vi "UHR-Fleezers Control (host) - 10.8MV_trial1.vi"() -> ()   [LabVIEW 2010] (continued)
    n1529 = Or(x=w5608, y=w5604) -> (x .or. y?=w5605:bool)
    n1530 = Square Root(x=w5388) -> (sqrt(x)=w5387:dbl)
    n1531 = Equal?(x="Tab Control 6", y=T37."High Res Display") -> (x = y?=w5528:bool)
    n1532 = Multiply(x="APD Disp. Scale", y=w5478) -> (x*y=w5487:waveform(dbl)[])
    n1533 = Multiply(x="APD Disp. Downsample", y=w5485) -> (x*y=w5483:dbl)
    n1534 = Multiply(x=10.0, y=w5387) -> (x*y=→"Trap 1 Position RMS (A)":dbl)
    n1535 = Divide(x=w5487, y=w5483) -> (x/y=w5455:waveform(dbl)[])
    n1536 = Index Array(array=w5455, index=0) -> (element=w5465:waveform(dbl))
    n1537 = case "For computing FFTs for display" shown="True" "Compute FFT" {
      tunnel: w5482 -> [_ w7808]
      frame False {
      }
      frame True {
        n1538 = Build Array("FFT 1 Choice 1", "FFT 1 Choice 2", "FFT 2 Choice 1", "FFT 2 Choice 2") -> (w7801:u16[])
        n1539 = Array Size(array=w7808) -> (size(s)=w7807:i32)
        n1540 = feedback-in #6(w7801) -> ()
        n1541 = feedback #6(u16[] [100, 100, 100, 100]) -> (w7802:u16[])
        n1542 = feedback-in #7("# Spectra to Ave.") -> ()
        n1543 = feedback #7("# Spectra to Ave.") -> (w7799:dbl)
        n1544 = Not Equal?(x="# Spectra to Ave.", y=w7799) -> (x != y?=w7798:bool)
        n1545 = Not Equal?(x=w7801, y=w7802) -> (x != y?=w7800:bool)
        n1546 = feedback #8(1.0) -> (w7785:dbl)
        n1547 = Compound Arithmetic op=OR("Reset FFT", w7800, w7798) -> (w7783:bool)
        n1548 = Select(t=1.0, s=w7783, f=w7785) -> (s? t:f=w7787:dbl)
        n1549 = Greater?(x=w7787, y="# Spectra to Ave.") -> (0:w7806:bool)
        n1550 = Increment(x=w7787) -> (x+1=w7786:dbl)
        n1551 = feedback-in #8(w7786) -> ()
        n1552 = local read "DMA Update Period (s)"() -> (w7781:dbl)
        n1553 = Multiply(x="# Spectra to Ave.", y=w7781) -> (x*y=→"Ave. Time (s)":dbl)
        n1554 = Build Array(cluster{"f0":dbl, "df":dbl, "magnitude":dbl[]} {"f0"=0.0, "df"=0.0, "magnitude"=[]} ("PSD")) -> (w7790:cluster{"f0":dbl, "df":dbl, "magnitude":dbl[]}[])
        n1555 = Build Array(w7790, w7790, w7790, w7790) -> (w7792:T49)
        n1556 = feedback #9(w7792) -> (w7797:T49)
        n1557 = for {
          N: 4 -> [_]
          tunnel: w7801 -> [w7830] mode=indexing
          tunnel: w7808 -> [w7831]
          tunnel: w7807 -> [w7833]
          tunnel: w7783 -> [w7826]
          tunnel: w7806 -> [w7825]
          tunnel: "# Spectra to Ave." -> [w7824]
          tunnel: [w7823] -> w7796 mode=indexing
          tunnel: w7797 -> [w7828] mode=indexing
          tunnel: [w7827] -> w7784 mode=indexing
          tunnel: w7787 -> [w7822]
          n1558 = Less?(x=w7830, y=w7833) -> (x < y?=w7832:bool)
          n1559 = Index Array(array=w7831, index=w7830) -> (element=w7829:waveform(dbl))
          n1560 = case shown="True" w7832 {
            tunnel: w7829 -> [_ w7850]
            tunnel: w7828 -> [w7835 w7848]
            tunnel: [w7835 w7836] -> w7827
            tunnel: w7826 -> [_ w7847]
            tunnel: w7825 -> [_ w7840]
            tunnel: w7824 -> [_ w7839]
            tunnel: [cluster{"f0":dbl, "df":dbl, "magnitude":dbl[]} {"f0"=0.0, "df"=0.0, "magnitude"=[]} ("PSD") w7841] -> w7823
            tunnel: w7822 -> [_ w7838]
            frame False {
            }
            frame True {
              n1561 = call <vilib>:"Std Deviation and Variance.vi"("X"=w7850) -> ("mean"=w7851:dbl)  [unwired: 1 in, 2 out]
              n1562 = Subtract(x=w7850, y=w7851) -> (x-y=w7849:waveform(dbl))
              n1563 = xnode "Spectral Measurements"("Signals"=w7849) -> ("PSD"=w7843:cluster{"f0":dbl, "df":dbl, "magnitude":dbl[]})  [unwired: 1 in, 1 out]
              n1564 = case shown="False" w7847 {
                tunnel: w7848 -> [w7860 _]
                tunnel: [w7856 w7865] -> w7836
                tunnel: w7843 -> [w7859 w7866]
                tunnel: w7840 -> [w7858 _]
                frame False {
                  n1565 = Build Array (concatenate)(w7860, w7859) -> (w7857:cluster{"f0":dbl, "df":dbl, "magnitude":dbl[]}[])
                  n1566 = case shown="True" w7858 {
                    tunnel: w7857 -> [w7861 w7864]
                    tunnel: [w7861 w7862] -> w7856
                    frame False {
                    }
                    frame True {
                      n1567 = Delete From Array(array=w7864, index=0) -> (array with subset deleted=w7862:cluster{"f0":dbl, "df":dbl, "magnitude":dbl[]}[])  [unwired: 1 in, 1 out]
                    }
                  }
                }
                frame True {
                  n1568 = Build Array(w7866) -> (w7865:cluster{"f0":dbl, "df":dbl, "magnitude":dbl[]}[])
                }
              }
              n1569 = for {
                tunnel: w7836 -> [w7855] mode=indexing
                tunnel: [w7854] -> w7846 mode=indexing
                workers-P: _ -> [_]
                n1570 = Unbundle By Name(w7855) -> ("magnitude"=w7854:dbl[])
              }
              n1571 = Transpose 2D Array(2D array=w7846) -> (transposed array=w7845:dbl[][])
              n1572 = for {
                tunnel: w7845 -> [w7853] mode=indexing
                tunnel: [w7852] -> w7844 mode=indexing
                workers-P: _ -> [_]
                n1573 = Add Array Elements(numeric array=w7853) -> (sum=w7852:dbl)
              }
              n1574 = Select(t=w7839, s=w7840, f=w7838) -> (s? t:f=w7837:dbl)
              n1575 = Divide(x=w7844, y=w7837) -> (x/y=w7842:dbl[])
              n1576 = Bundle By Name(cluster=w7843, "magnitude"=w7842) -> (w7841:cluster{"f0":dbl, "df":dbl, "magnitude":dbl[]})
            }
          }
        }
        n1577 = case shown="True" w7783 {
          tunnel: w7784 -> [w7815 w7821]
          tunnel: [w7815 w7816] -> w7782
          frame False {
          }
          frame True {
            n1578 = Array Subset(array=w7821, index (row)=0 ("index"), length (row)=4 ("length"), index (col)=0 ("index"), length (col)=1 ("length")) -> (w7816:T49)
          }
        }
        n1579 = feedback-in #9(w7782) -> ()
        n1580 = Split 1D Array(array=w7796, index=2) -> (first subarray=→"FFT 1":cluster{"f0":dbl, "df":dbl, "magnitude":dbl[]}[], second subarray=→"FFT 2":cluster{"f0":dbl, "df":dbl, "magnitude":dbl[]}[])
      }
    }
    n1581 = Index Array(array=w5455, index=1) -> (element=w5463:waveform(dbl))
    n1582 = case "For displaying the high resolution display (no downsampling)" shown="True" w5528 {
      tunnel: w5482 -> [_ w5990]
      frame False {
      }
      frame True {
        n1583 = Index Array(array=w5990, index="High Res. Display") -> (element=w5991:waveform(dbl))
        n1584 = call <vilib>:"Std Deviation and Variance.vi"("X"=w5991) -> ("mean"=w5998:dbl, "standard deviation"=w6003:dbl)  [unwired: 1 in, 1 out]
        "Mean Intensity" <- w5998
        "Sigma" <- w6003
        n1585 = Subtract(x=w5991, y=w5998) -> (x-y=w5997:waveform(dbl))
        n1586 = Select(t=w5997, s="Subtract mean", f=w5991) -> (s? t:f=→"1 Channel":waveform(dbl))
        n1587 = Divide(x=w6003, y=w5998) -> (x/y=→"Sigma/Mean":dbl)
        n1588 = feedback #10(1) -> (w5992:i32)
        n1589 = Greater Or Equal?(x=w5992, y="Slow mean N ave.") -> (x >= y?=w6005:bool)
        n1590 = Increment(x=w5992) -> (x+1=w6007:i32)
        n1591 = Select(t=1, s=w6005, f=w6007) -> (s? t:f=w5994:i32)
        n1592 = feedback-in #10(w5994) -> ()
        n1593 = feedback #11() -> (w5995:waveform(dbl))  [unwired: 1 out]
        n1594 = case shown="Default" w5992 {
          tunnel: [w6010 w6013] -> w5996
          tunnel: w5995 -> [w6012 _]
          tunnel: w5991 -> [w6011 w6013]
          frame Default {
            n1595 = call-poly <vilib>:"Append Waveforms.vi"("waveform B"=w6011, "waveform A"=w6012) -> ("waveform out"=w6010:waveform(dbl))  [unwired: 1 in, 8 out]
          }
          frame 1 {
          }
        }
        n1596 = feedback-in #11(w5996) -> ()
        n1597 = case shown="True" w6005 {
          tunnel: w5996 -> [_ w6009]
          frame False {
          }
          frame True {
            n1598 = call <vilib>:"Mean.vi"("X"=w6009) -> ("mean"=→"Slow mean":dbl)  [unwired: 1 out]
          }
        }
      }
    }
    n1599 = case "For plotting results of scanning MCL" shown="True" w5605 {
      tunnel: w5604 -> [_ w6521]
      tunnel: w5521 -> [_ w6617]
      tunnel: w5613 -> [_ _]
      tunnel: w5482 -> [_ w6591]
      tunnel: w5457 -> [_ w6522]
      tunnel: w5456 -> [_ w6495]
      frame False {
      }
      frame True {
        w6502 = u32 0 items=["Horizontal", "Vertical", "Central", "1st Diagonal", "2nd Diagonal"] ("Type of Symmetry")
        w6530 = u32 0 items=["Horizontal", "Vertical", "Central", "1st Diagonal", "2nd Diagonal"] ("Type of Symmetry")
        w6533 = u32 0 items=["Horizontal", "Vertical", "Central", "1st Diagonal", "2nd Diagonal"] ("Type of Symmetry")
        w6562 = u32 0 items=["Horizontal", "Vertical", "Central", "1st Diagonal", "2nd Diagonal"] ("Type of Symmetry")
        n1600 = Index Array(array=w6591, index=10) -> (element=w6597:waveform(dbl))
        n1601 = Index Array(array=w6591, index=11) -> (element=w6594:waveform(dbl))
        n1602 = local read "Cycles/step (MCL)"() -> (w6547:u64)
        n1603 = Index Array(array=w6591, index="Channel") -> (element=w6593:waveform(dbl))
        n1604 = Unbundle(w6495) -> ("New Image"=w6494:T2, "New Image"=w6493:T2, "New Image"=w6492:T2, "New Image"=w6491:T2)
        n1605 = Unbundle By Name(w6597) -> ("Y"=w6549:dbl[])
        n1606 = Unbundle By Name(w6594) -> ("Y"=w6551:dbl[])
        n1607 = Unbundle By Name(w6593) -> ("Y"=w6556:dbl[])
        n1608 = call "downsample 1D array - double.vi"("Ave N"=w6547, "Array In"=w6549) -> ("Array Out"=w6548:dbl[])  [unwired: 1 out]
        n1609 = call "downsample 1D array - double.vi"("Ave N"=w6547, "Array In"=w6551) -> ("Array Out"=w6550:dbl[])  [unwired: 1 out]
        n1610 = call "downsample 1D array - double.vi"("Ave N"=w6547, "Array In"=w6556) -> ("Array Out"=w6555:dbl[])  [unwired: 1 out]
        n1611 = feedback #12(w6617) -> (w6618:dbl[])
        n1612 = Build Array (concatenate)(w6618, w6617) -> (w6599:dbl[])
        n1613 = feedback #13(w6522) -> (w6524:dbl[])
        n1614 = Build Array (concatenate)(w6524, w6522) -> (w6523:dbl[])
        n1615 = local read "Scan steps (MCL)"() -> (w6504:u64)
        n1616 = Select(t=w6617, s=w6521, f=w6599) -> (s? t:f=w6603:dbl[])
        n1617 = feedback-in #12(w6603) -> ()
        n1618 = Select(t=w6522, s=w6521, f=w6523) -> (s? t:f=w6505:dbl[])
        n1619 = feedback-in #13(w6505) -> ()
        n1620 = local read "Scan lines (y)"() -> (w6490:u64)
        n1621 = local read "N APD Samp/step"() -> (w6506:dbl)
        n1622 = feedback #14(w6548) -> (w6605:dbl[])
        n1623 = Build Array (concatenate)(w6605, w6548) -> (w6596:dbl[])
        n1624 = feedback #15(w6555) -> (w6615:dbl[])
        n1625 = Build Array (concatenate)(w6615, w6555) -> (w6614:dbl[])
        n1626 = feedback #16(w6550) -> (w6607:dbl[])
        n1627 = Build Array (concatenate)(w6607, w6550) -> (w6608:dbl[])
        n1628 = Select(t=w6548, s=w6521, f=w6596) -> (s? t:f=w6552:dbl[])
        n1629 = feedback-in #14(w6552) -> ()
        n1630 = Select(t=w6555, s=w6521, f=w6614) -> (s? t:f=w6554:dbl[])
        n1631 = feedback-in #15(w6554) -> ()
        n1632 = Select(t=w6550, s=w6521, f=w6608) -> (s? t:f=w6553:dbl[])
        n1633 = feedback-in #16(w6553) -> ()
        n1634 = Multiply(x=w6504, y=u64 2) -> (x*y=w6489:u64)
        n1635 = call "integrate 1D array interval - double.vi"("Ave N"=w6506, "Array In"=w6505) -> ("Array Out"=w6517:dbl[])  [unwired: 1 out]
        n1636 = call "integrate 1D array interval - double.vi"("Ave N"=w6506, "Array In"=w6603) -> ("Array Out"=w6602:dbl[])  [unwired: 1 out]
        n1637 = Array Size(array=w6517) -> (size(s)=w6518:i32)
        n1638 = Array Size(array=w6602) -> (size(s)=w6604:i32)
        n1639 = Multiply(x=w6490, y=w6489) -> (x*y=w6520:u64)
        n1640 = Multiply(x=w6490, y=w6489) -> (x*y=w6612:u64)
        n1641 = call <vilib>:"Mean.vi"("X"=w6552) -> ("mean"=w6536:dbl)  [unwired: 1 out]
        n1642 = Subtract(x=w6520, y=w6518) -> (x-y=w6511:u64)
        n1643 = call <vilib>:"Mean.vi"("X"=w6554) -> ("mean"=w6541:dbl)  [unwired: 1 out]
        n1644 = call <vilib>:"Mean.vi"("X"=w6553) -> ("mean"=w6539:dbl)  [unwired: 1 out]
        n1645 = call <vilib>:"Mean.vi"("X"=w6517) -> ("mean"=w6508:dbl)  [unwired: 1 out]
        n1646 = Subtract(x=w6612, y=w6604) -> (x-y=w6546:u64)
        n1647 = call <vilib>:"Mean.vi"("X"=w6602) -> ("mean"=w6543:dbl)  [unwired: 1 out]
        n1648 = Initialize Array(1.0 ("element"), w6511) -> (w6507:dbl[])
        n1649 = Initialize Array(1.0 ("element"), w6546) -> (w6537:dbl[])
        n1650 = Multiply(x=w6507, y=w6508) -> (x*y=w6509:dbl[])
        n1651 = Multiply(x=w6537, y=w6539) -> (x*y=w6540:dbl[])
        n1652 = Multiply(x=w6537, y=w6541) -> (x*y=w6542:dbl[])
        n1653 = Multiply(x=w6537, y=w6536) -> (x*y=w6538:dbl[])
        n1654 = Multiply(x=w6537, y=w6543) -> (x*y=w6544:dbl[])
        n1655 = Build Array (concatenate)(w6552, w6538) -> (w6606:dbl[])
        n1656 = Build Array (concatenate)(w6554, w6542) -> (w6610:dbl[])
        n1657 = Build Array (concatenate)(w6553, w6540) -> (w6609:dbl[])
        n1658 = Build Array (concatenate)(w6517, w6509) -> (w6519:dbl[])
        n1659 = Build Array (concatenate)(w6602, w6544) -> (w6611:dbl[])
        n1660 = Reshape Array(w6606, w6490, w6489) -> (w6572:dbl[][])
        n1661 = Reshape Array(w6519, w6490, w6489) -> (w6515:dbl[][])
        n1662 = Reshape Array(w6610, w6490, w6489) -> (w6564:dbl[][])
        n1663 = Reshape Array(w6609, w6490, w6489) -> (w6579:dbl[][])
        n1664 = Reshape Array(w6611, w6490, w6489) -> (w6589:dbl[][])
        n1665 = Array Subset(array=w6579, index (col)=0 ("index"), length (col)=w6504) -> (w6584:dbl[][])  [unwired: 2 in]
        n1666 = Array Subset(array=w6579, index (col)=w6504) -> (w6582:dbl[][])  [unwired: 3 in]
        n1667 = Array Subset(array=w6564, index (col)=0 ("index"), length (col)=w6504) -> (w6570:dbl[][])  [unwired: 2 in]
        n1668 = Array Subset(array=w6564, index (col)=w6504) -> (w6568:dbl[][])  [unwired: 3 in]
        n1669 = Array Subset(array=w6515, index (col)=0 ("index"), length (col)=w6504) -> (w6514:dbl[][])  [unwired: 2 in]
        n1670 = Array Subset(array=w6515, index (col)=w6504) -> (w6512:dbl[][])  [unwired: 3 in]
        n1671 = Array Subset(array=w6589, index (col)=0 ("index"), length (col)=w6504) -> (w6588:dbl[][])  [unwired: 2 in]
        n1672 = Array Subset(array=w6589, index (col)=w6504) -> (w6586:dbl[][])  [unwired: 3 in]
        n1673 = Array Subset(array=w6572, index (col)=0 ("index"), length (col)=w6504) -> (w6577:dbl[][])  [unwired: 2 in]
        n1674 = Array Subset(array=w6572, index (col)=w6504) -> (w6575:dbl[][])  [unwired: 3 in]
        n1675 = for {
          tunnel: w6584 -> [w6626] mode=indexing
          tunnel: [w6625] -> w6583 mode=indexing
          workers-P: _ -> [_]
          n1676 = Reverse 1D Array(array=w6626) -> (reversed array=w6625:dbl[])
        }
        n1677 = for {
          tunnel: w6570 -> [w6622] mode=indexing
          tunnel: [w6621] -> w6569 mode=indexing
          workers-P: _ -> [_]
          n1678 = Reverse 1D Array(array=w6622) -> (reversed array=w6621:dbl[])
        }
        n1679 = for {
          tunnel: w6514 -> [w6620] mode=indexing
          tunnel: [w6619] -> w6513 mode=indexing
          workers-P: _ -> [_]
          n1680 = Reverse 1D Array(array=w6620) -> (reversed array=w6619:dbl[])
        }
        n1681 = for {
          tunnel: w6588 -> [w6628] mode=indexing
          tunnel: [w6627] -> w6587 mode=indexing
          workers-P: _ -> [_]
          n1682 = Reverse 1D Array(array=w6628) -> (reversed array=w6627:dbl[])
        }
        n1683 = for {
          tunnel: w6577 -> [w6624] mode=indexing
          tunnel: [w6623] -> w6576 mode=indexing
          workers-P: _ -> [_]
          n1684 = Reverse 1D Array(array=w6624) -> (reversed array=w6623:dbl[])
        }
        n1685 = Index Array(array=w6589, index (row)=0) -> (element=→"Waveform Graph":dbl[])  [unwired: 1 in]
        n1686 = Add(x=w6583, y=w6582) -> (x+y=w6581:dbl[][])
        n1687 = Add(x=w6569, y=w6568) -> (x+y=w6567:dbl[][])
        n1688 = Add(x=w6513, y=w6512) -> (x+y=w6497:dbl[][])
        n1689 = Add(x=w6587, y=w6586) -> (x+y=w6561:dbl[][])
        n1690 = Add(x=w6576, y=w6575) -> (x+y=w6574:dbl[][])
        n1691 = Divide(x=w6567, y=2) -> (x/y=w6565:dbl[][])
        n1692 = Divide(x=w6581, y=2) -> (x/y=w6526:dbl[][])
        n1693 = Divide(x=w6574, y=2) -> (x/y=w6528:dbl[][])
        n1694 = To Single Precision Float(number=w6561) -> (single precision float=w6560:sgl[][])
        n1695 = Transpose 2D Array(2D array=w6565) -> (transposed array=→"Data map":dbl[][])
        n1696 = To Single Precision Float(number=w6497) -> (single precision float=w6501:sgl[][])
        n1697 = To Single Precision Float(number=w6526) -> (single precision float=w6532:sgl[][])
        n1698 = To Single Precision Float(number=w6528) -> (single precision float=w6529:sgl[][])
        n1699 = call "IMAQ ArrayToImage"("Image Pixels (Float)"=w6560, "Image"=w6494) -> ("Image Out"=w6563:T2)  [unwired: 8 in, 1 out]
        n1700 = call "IMAQ ArrayToImage"("Image Pixels (Float)"=w6501, "Image"=w6493) -> ("Image Out"=w6503:T2)  [unwired: 8 in, 1 out]
        n1701 = call "IMAQ ArrayToImage"("Image Pixels (Float)"=w6532, "Image"=w6492) -> ("Image Out"=w6534:T2)  [unwired: 8 in, 1 out]
        n1702 = call "IMAQ ArrayToImage"("Image Pixels (Float)"=w6529, "Image"=w6491) -> ("Image Out"=w6531:T2)  [unwired: 8 in, 1 out]
        n1703 = call "IMAQ Symmetry"("Type of Symmetry"=w6562, "Image Src"=w6563) -> ("Image Dst Out"=w6558:T2)  [unwired: 3 in, 1 out]
        n1704 = call "IMAQ Symmetry"("Type of Symmetry"=w6502, "Image Src"=w6503) -> ("Image Dst Out"=w6499:T2)  [unwired: 3 in, 1 out]
        n1705 = call "IMAQ Symmetry"("Type of Symmetry"=w6533, "Image Src"=w6534) -> ("Image Dst Out"=→"Detection Laser X":T2)  [unwired: 3 in, 1 out]
        n1706 = call "IMAQ Symmetry"("Type of Symmetry"=w6530, "Image Src"=w6531) -> ("Image Dst Out"=→"Detection Laser Y":T2)  [unwired: 3 in, 1 out]
        n1707 = call "IMAQ Set Simple Calibration"("Calibration Axis Info"=T38 {"Origin Pixel"={"X"=0.0, "Y"=0.0}, "Angle Relative to Horizontal (deg)"=0.0, "Axis Reference"=0}, "Grid Descriptor"=T39 {"X Step"=0.3, "Y Step"=0.3, "Unit"=enum."Undefined"}, "Image"=w6558) -> ("Calibrated Image"=→"APD 1":T2)  [unwired: 7 in, 1 out]
        n1708 = call "IMAQ Set Simple Calibration"("Calibration Axis Info"=T38 {"Origin Pixel"={"X"=0.0, "Y"=0.0}, "Angle Relative to Horizontal (deg)"=0.0, "Axis Reference"=0}, "Grid Descriptor"=T39 {"X Step"=0.3, "Y Step"=0.3, "Unit"=enum."Undefined"}, "Image"=w6499) -> ("Calibrated Image"=→"APD 2":T2)  [unwired: 7 in, 1 out]
      }
    }
    n1709 = Subtract(x=w5463, y="APD 2 Offset") -> (x-y=w5460:waveform(dbl))
    n1710 = Subtract(x=w5465, y="APD 1 Offset") -> (x-y=w5461:waveform(dbl))
    n1711 = Index Array(array=w5480, index=3) -> (element=w5549:waveform(dbl))
    n1712 = Index Array(array=w5480, index=6) -> (element=w5546:waveform(dbl))
    n1713 = Build Array(w5461, w5460) -> (→"APD Chart":waveform(dbl)[])
    n1714 = Array Size(array=w5538) -> (size(s)=w5593:i32)
    n1715 = call <vilib>:"Std Deviation and Variance.vi"("X"=w5473) -> ("standard deviation"=w5472:dbl)  [unwired: 1 in, 2 out]
    n1716 = Add Array Elements(numeric array=w5473) -> (sum=w5475:u32)
    n1717 = Add Array Elements(numeric array=w5538) -> (sum=w5603:u32)
    n1718 = call <vilib>:"Std Deviation and Variance.vi"("X"=w5538) -> ("standard deviation"=w5537:dbl)  [unwired: 1 in, 2 out]
    n1719 = Divide(x="T1 offset_x (mV)", y=1000.0) -> (x/y=w5550:dbl)
    n1720 = Divide(x=w5472, y=w5471) -> (x/y=w5468:dbl)
    "Rate sigma (Hz) 2" <- w5468
    n1721 = Multiply(x=w5471, y=w5593) -> (x*y=w5474:dbl)
    "Int. Time (s)" <- w5474
    n1722 = Divide(x=w5475, y=w5474) -> (x/y=w5469:dbl)
    "APD 2 Rate (Hz)" <- w5469
    n1723 = Divide(x=w5603, y=w5474) -> (x/y=w5535:dbl)
    "APD 1 Rate (Hz)" <- w5535
    n1724 = Divide(x=w5537, y=w5471) -> (x/y=w5536:dbl)
    "Rate sigma (Hz)" <- w5536
    n1725 = Divide(x=w5468, y=w5469) -> (x/y=→"Sigma/Mean 2":dbl)
    n1726 = Divide(x=w5536, y=w5535) -> (x/y=→"Sigma/Mean":dbl)
    n1727 = Divide(x="T2 offset_x (mV)", y=1000.0) -> (x/y=w5548:dbl)
    n1728 = case shown="1" "Calibration" {
      tunnel: "T1 alpha_x (nm/V)" -> [_ w6457 w6478]
      tunnel: "T1 kappa_x (pN/nm)" -> [_ _ w6468]
      tunnel: "T2 alpha_x (nm/V)" -> [_ w6456 w6476]
      tunnel: "T2 kappa_x (pN/nm)" -> [_ _ w6469]
      tunnel: w5549 -> [w6439 w6454 w6474]
      tunnel: w5546 -> [w6438 w6452 w6472]
      tunnel: [w6439 w6451 w6471] -> w5579
      tunnel: [w6438 w6450 w6470] -> w5578
      tunnel: ["T1 X (V)" ("Label.Text") "T1 X (nm)" ("Label.Text") "T1 X (pN)" ("Label.Text")] -> w5567
      tunnel: ["T2 X (V)" ("Label.Text") "T2 X (nm)" ("Label.Text") "T2 X (pN)" ("Label.Text")] -> w5566
      tunnel: ["Position (V)" ("Label.Text") "Position (nm)" ("Label.Text") "Force (pN)" ("Label.Text")] -> w5568
      tunnel: w5548 -> [_ w6442 w6461]
      tunnel: w5550 -> [_ w6445 w6463]
      tunnel: ["Mean (V)" ("Label.Text") "Mean (nm)" ("Label.Text") "Mean (pN)" ("Label.Text")] -> w5563
      tunnel: ["Difference (V)" ("Label.Text") "Difference (nm)" ("Label.Text") "Difference (pN)" ("Label.Text")] -> w5488
      frame 0, Default {
      }
      frame 1 {
        # "position"
        n1729 = Unbundle By Name(w6454) -> ("Y"=w6458:dbl[])
        n1730 = Unbundle By Name(w6452) -> ("Y"=w6443:dbl[])
        n1731 = Subtract(x=w6458, y=w6445) -> (x-y=w6446:dbl[])
        n1732 = Subtract(x=w6443, y=w6442) -> (x-y=w6444:dbl[])
        n1733 = Multiply(x=w6444, y=w6456) -> (x*y=w6453:dbl[])
        n1734 = Multiply(x=w6457, y=w6446) -> (x*y=w6455:dbl[])
        n1735 = Bundle By Name(cluster=w6452, "Y"=w6453) -> (w6450:waveform(dbl))
        n1736 = Bundle By Name(cluster=w6454, "Y"=w6455) -> (w6451:waveform(dbl))
      }
      frame 2 {
        # "force"
        n1737 = Unbundle By Name(w6474) -> ("Y"=w6479:dbl[])
        n1738 = Unbundle By Name(w6472) -> ("Y"=w6477:dbl[])
        n1739 = Subtract(x=w6477, y=w6461) -> (x-y=w6462:dbl[])
        n1740 = Subtract(x=w6479, y=w6463) -> (x-y=w6464:dbl[])
        n1741 = Compound Arithmetic op=MULTIPLY(w6462, w6476, w6469) -> (w6473:dbl[])
        n1742 = Compound Arithmetic op=MULTIPLY(w6468, w6478, w6464) -> (w6475:dbl[])
        n1743 = Bundle By Name(cluster=w6472, "Y"=w6473) -> (w6470:waveform(dbl))
        n1744 = Bundle By Name(cluster=w6474, "Y"=w6475) -> (w6471:waveform(dbl))
      }
    }
    n1745 = feedback-in #17("Calibration") -> ()
    n1746 = feedback #17(u16 1 ("Calibration")) -> (w5570:u16)
    n1747 = Not Equal?(x=w5570, y="Calibration") -> (x != y?=w5526:bool)
    n1748 = Unbundle By Name(w5549) -> ("Y"=w5552:dbl[])
    n1749 = Unbundle By Name(w5546) -> ("Y"=w5555:dbl[])
    n1750 = Subtract(x=w5552, y=w5550) -> (x-y=w5553:dbl[])
    n1751 = Subtract(x=w5555, y=w5548) -> (x-y=w5554:dbl[])
    n1752 = disable-structure shown="Enabled" {
      disable-tunnel: [-1.0 ("y") 1.0] -> w5556
      frame Disabled {
      }
      frame Enabled {
      }
    }
    n1753 = Multiply(x=w5554, y="T2 alpha_x (nm/V)") -> (x*y=w5545:dbl[])
    n1754 = Multiply(x="T1 alpha_x (nm/V)", y=w5553) -> (x*y=w5544:dbl[])
    n1755 = Multiply(x=w5578, y=w5556) -> (x*y=w5557:waveform(dbl))
    n1756 = case shown="True" "Read Lateness and Rel Phase" {
      tunnel: w5380 -> [w6014 w6036]
      tunnel: w5379 -> [w6015 w6035]
      tunnel: [w6014 w6034] -> w5541
      tunnel: [w6015 w6033] -> w5540
      frame False {
      }
      frame True {
        n1757 = xnode "Read/Write Control"("FPGA VI Reference In"=w6036, "error in"=w6035) -> ("FPGA VI Reference Out"=w6034:T19, "error out"=w6033:errorcluster, "GI Relative phase"=→"GI relative phase":i16, "Relative phase"=→"Relative phase (AI1)":i16, "AI Late Counter"=→"Late Counter (AI1)":u16, "GI Late Counter"=→"GI Late Counter":u16, "MCL Late Counter"=→"MCL Late Counter":u16, "MCL Relative Phase"=→"Relative Phase (MCL)":i16, "APD Acq Relative Phase"=→"APD Acq Relative Phase":i16, "APD 1 Gate Relative Phase"=→"APD 1 Gate Relative Phase":i16, "APD 2 Gate Relative Phase"=→"APD 2 Gate Relative Phase":i16, "APD Acq Late Counter"=→"APD Acq Late Counter":u16, "APD 1 Gate Late Counter"=→"APD 1 Gate Late Counter":u16, "APD 2 Gate Late Counter"=→"APD 2 Gate Late Counter":u16, "Green FB Relative Phase"=→"Relative phase (Green FB)":i16, "GI Relative phase 2"=→"GI relative phase 2":i16, "GI Late Counter 2"=→"GI Late Counter 2":u16, "Trap Pos FIFO Timeout"=→"Trap Pos FIFO Timeout":u16, "Trap AI FIFO Timeout"=→"Trap AI FIFO Timeout":u16)
      }
    }
    n1758 = Subtract(x=w5545, y=w5544) -> (x-y=w5543:dbl[])
    n1759 = Unbundle By Name(w5578) -> ("Y"=w5513:dbl[])
    n1760 = Unbundle By Name(w5579) -> ("Y"=w5514:dbl[])
    n1761 = Build Array(w5579, w5557) -> (→"Force":waveform(dbl)[])
    n1762 = Subtract(x=w5543, y="Offset (nm)") -> (x-y=w5511:dbl[])
    n1763 = call <vilib>:"Mean.vi"("X"=w5513) -> ("mean"=w5492:dbl)  [unwired: 1 out]
    "T2 X" <- w5492
    n1764 = Absolute Value(x=w5514) -> (abs(x)=w5515:dbl[])
    n1765 = Absolute Value(x=w5513) -> (abs(x)=w5516:dbl[])
    n1766 = call <vilib>:"Mean.vi"("X"=w5514) -> ("mean"=w5493:dbl)  [unwired: 1 out]
    "T1 X" <- w5493
    n1767 = Add(x=w5515, y=w5516) -> (x+y=w5517:dbl[])
    n1768 = Bundle By Name(cluster=w5549, "Y"=w5511) -> (w5479:waveform(dbl))
    "Bead Separation" <- w5479
    n1769 = Divide(x=w5517, y=2.0) -> (x/y=→"Vec Mean of T1 T2":dbl[])
    n1770 = case shown="True" w5526 {
      tunnel: w5568 -> [_ w6432]
      tunnel: w5567 -> [_ w6431]
      tunnel: w5566 -> [_ w6430]
      tunnel: w5563 -> [_ w6429]
      tunnel: w5488 -> [_ w6428]
      frame False {
      }
      frame True {
        n1771 = property on="Force" class="WFChart (strict)"("YScale.NameLbl.Text"=w6432) -> ()  [unwired: 2 in, 2 out]
        n1772 = property on="T2 X" class="DigNum (strict)"("Caption.Text"=w6430) -> ()  [unwired: 2 in, 2 out]
        n1773 = property on="T1 X" class="DigNum (strict)"("Caption.Text"=w6431) -> ()  [unwired: 2 in, 2 out]
        n1774 = property on="Mean" class="DigNum (strict)"("Caption.Text"=w6429) -> ()  [unwired: 2 in, 2 out]
        n1775 = property on="Difference" class="DigNum (strict)"("Caption.Text"=w6428) -> ()  [unwired: 2 in, 2 out]
      }
    }
    n1776 = local read "Tether"() -> (w5520:bool)
    n1777 = Absolute Value(x=w5493) -> (abs(x)=w5490:dbl)
    n1778 = Absolute Value(x=w5492) -> (abs(x)=w5489:dbl)
    n1779 = Add(x=w5490, y=w5489) -> (x+y=w5565:dbl)
    n1780 = Subtract(x=w5490, y=w5489) -> (x-y=→"Difference":dbl)
    n1781 = feedback #18(w5511) -> (w5510:dbl[])
    n1782 = Divide(x=w5565, y=2.0) -> (x/y=w5519:dbl)
    "Mean" <- w5519
    n1783 = case shown="True" w5520 {
      tunnel: w5519 -> [_ w5973]
      frame False {
      }
      frame True {
        n1784 = Greater?(x="Lost Tether Alarm Threshold (pN)", y=w5973) -> (0:w5971:bool)
        n1785 = case shown="True" w5971 {
          frame False {
          }
          frame True {
            n1786 = flat-sequence {
              frame #0 {
                # "stop only if saving"
                n1787 = local read "Saving..."() -> (w5986:bool)
                n1788 = And(x=w5986, y="TA Cancel Save?") -> (x .and. y?=w5985:bool)
                n1789 = local write "Stop Saving"(w5985) -> ()
              }
              frame #1 {
                n1790 = case shown="True" "TA Green Off?" {
                  frame False {
                  }
                  frame True {
                    w5989 = FALSE ("Fl. Triggered...")
                    n1791 = local write "Fl. Triggered..."(w5989) -> ()
                    n1792 = property on="Green Laser ON/Interlacing" class="Bool (strict)"("Val(Sgnl)"=w5989) -> ()  [unwired: 2 in, 2 out]
                  }
                }
              }
            }
            n1793 = local read "Time tether formed"() -> (w5980:timestamp)
            n1794 = Get Date/Time In Seconds() -> (seconds since 1Jan1904=w5981:timestamp)
            n1795 = Subtract(x=w5981, y=w5980) -> (x-y=w5979:dbl)
            n1796 = Number To Decimal String(number=w5979) -> (decimal integer string=w5976:string)  [unwired: 1 out]
            n1797 = local read "Messages"() -> (w5983:string)
            n1798 = call <vilib>:"Beep.vi"() -> ()  [unwired: 3 in, 9 out]
            n1799 = Concatenate Strings("Lost tether (" ("Message to add"), w5976, " s)." ("string")) -> (w5978:string)
            n1800 = local write "Tether"(FALSE ("Tether")) -> ()
            n1801 = call "Update messages.vi"("Message to add"=w5978, "Old message string"=w5983) -> ("New message string"=w5982:string)
            n1802 = local write "Messages"(w5982) -> ()
            n1803 = property on="Trap Pos. FB ON" class="Bool (strict)"("Val(Sgnl)"=FALSE ("Value (Signaling)")) -> ()  [unwired: 2 in, 2 out]
          }
        }
      }
    }
    n1804 = Build Array (concatenate)(w5511, w5510) -> (w5509:dbl[])
    n1805 = Split 1D Array(array=w5509, index=w5391) -> (first subarray=w5505:dbl[])  [unwired: 1 out]
    n1806 = feedback-in #18(w5505) -> ()
    n1807 = call <vilib>:"Mean.vi"("X"=w5505) -> ("mean"=w5504:dbl)  [unwired: 1 out]
    "Bead Mean (nm)" <- w5504
    n1808 = Subtract(x=w5505, y=w5504) -> (x-y=w5503:dbl[])
    n1809 = Square(x=w5503) -> (x^2=w5502:dbl[])
    n1810 = call <vilib>:"Mean.vi"("X"=w5502) -> ("mean"=w5501:dbl)  [unwired: 1 out]
    n1811 = Square Root(x=w5501) -> (sqrt(x)=w5500:dbl)
    n1812 = Multiply(x=10.0, y=w5500) -> (x*y=→"RMS (Ang)":dbl)
    n1813 = xnode "Read/Write Control"("FPGA VI Reference In"=w5541, "error in"=w5540) -> ("FPGA VI Reference Out"=w5659:T19, "error out"=w5653:errorcluster, "AI2 Y Sum Set 1"=w5649:i16, "AI2 Y Sum Set 2"=w5648:i16, "AI1 X Set 1"=w5425:fxp<+/-,16,1>, "AI1 X Set 2"=w5424:fxp<+/-,16,1>, "Trap Pos FB Int Signal"=→"Trap Pos FB Int Signal":fxp<+/-,24,9>, "Trap Pos FB Int-Norm Signal"=→"Trap Pos FB Int-Norm Signal":fxp<+/-,16,1>, "Trap Pos FB Action"=w5418:i64, "Scanning"=→"AOD Scanning":bool, "Scan I"=→"AOD Scan I":u64, "Scanning MCL"=w5651:bool, "Scan I (MCL)"=→"MCL Scan I":u64, "Green FB Signals"=w5588:T43)  [unwired: 1 out]
    "MCL Scanning" <- w5651
    "Trap Pos FB Action" <- w5418
    n1814 = local read "AI2 (V)"() -> (w5650:cluster{"Set 1":dbl, "Set 2":dbl})
    n1815 = Bundle By Name(cluster=w5650, "Set 1"=w5649, "Set 2"=w5648) -> (w5646:cluster{"Set 1":dbl, "Set 2":dbl})
    n1816 = Divide(x=w5418, y=327.67) -> (x/y=→"Action (%)":dbl)
    n1817 = local read "Trap X (AI1)"() -> (w5438:T10)
    n1818 = Divide(x=w5646, y=3276.7) -> (x/y=w5645:cluster{"Set 1":dbl, "Set 2":dbl})
    n1819 = local write "AI2 (V)"(w5645) -> ()
    n1820 = Bundle(cluster=w5438, "Trap 1"=w5425, "Trap 2"=w5424) -> (→"Trap X (AI1)":T10)
    n1821 = Divide(x=w5588, y=3276.7) -> (x/y=w5584:T50)
    n1822 = Unbundle By Name(w5584) -> ("Green FB Ch 0"=w5587:dbl, "Green FB Ch 1"=w5586:dbl, "Green FB Ch 2"=w5585:dbl)
    n1823 = Divide(x=w5587, y=w5585) -> (x/y=w5583:dbl)
    n1824 = Divide(x=w5586, y=w5585) -> (x/y=w5582:dbl)
    n1825 = flat-sequence "To save data" {
      tunnel: [w8289] -> w5670
      tunnel: [w8290] -> w5669
      tunnel: w5619 -> [w8283]
      tunnel: w5507 -> [w8287]
      tunnel: ["Save Calibration"] -> w5642
      tunnel: w5639 -> [w8286]
      tunnel: [w8279] -> w5638
      tunnel: [w8276] -> w5637
      tunnel: [w8273] -> w5636
      tunnel: w5618 -> [w8275]
      tunnel: w5524 -> [w8269]
      tunnel: [w8269] -> w5523
      tunnel: ["Start Saving"] -> w5481
      tunnel: [w8263] -> w5407
      tunnel: [w8262] -> w5406
      tunnel: w5670 -> [w8524]
      tunnel: w5669 -> [w8523]
      tunnel: w5408 -> [w8522]
      tunnel: w5642 -> [w8521]
      tunnel: w5638 -> [w8519]
      tunnel: w5637 -> [w8518]
      tunnel: w5636 -> [w8517]
      tunnel: w5494 -> [w8516]
      tunnel: w5533 -> [w8515]
      tunnel: w5523 -> [w8514]
      tunnel: w5481 -> [w8513]
      tunnel: w5479 -> [w8512]
      tunnel: w5455 -> [w8511]
      tunnel: w5407 -> [w8510]
      tunnel: w5406 -> [w8509]
      tunnel: w5405 -> [w8508]
      frame #0 {
        n1826 = Or(x="Save N Sets", y="Start Saving") -> (x .or. y?=w8270:bool)
        n1827 = To Double Precision Float(number=w8286) -> (double precision float=w8280:dbl)
        n1828 = Build Array(w8270, "Save Calibration", w8283, w8275) -> (w8285:bool[])
        n1829 = Compound Arithmetic op=OR("Save Calibration", w8283, w8270, w8275) -> (w8288:bool)
        n1830 = Boolean Array To Number(Boolean array=w8285) -> (number=w8282:u32)
        n1831 = feedback #19(FALSE ("Save APD Data\nwith Trap Data")) -> (w8264:bool)
        n1832 = feedback #20(refnum<k0> refnum) -> (w8291:refnum<file>)
        n1833 = feedback #21(refnum<k0> refnum) -> (w8266:refnum<file>)
        n1834 = feedback #22(FALSE ("Save APD Data\nwith Trap Data")) -> (w8274:bool)
        n1835 = feedback #23(refnum<k0> refnum) -> (w8277:refnum<file>)
        n1836 = feedback #24(0) -> (w8293:i32)
        n1837 = feedback #25() -> (w8281:u32)  [unwired: 1 out]
        n1838 = case shown="True" w8288 {
          tunnel: [w8300 1] -> w8289
          tunnel: w8293 -> [w8302 _]
          tunnel: [w8301 w8320] -> w8290
          tunnel: w8291 -> [w8301 _]
          tunnel: w8287 -> [_ w8340]
          tunnel: w8280 -> [_ w8338]
          tunnel: w8282 -> [_ w8341]
          tunnel: [w8299 w8319] -> w8279
          tunnel: w8281 -> [w8299 _]
          tunnel: [w8298 w8317] -> w8276
          tunnel: w8277 -> [w8298 _]
          tunnel: [w8297 w8316] -> w8273
          tunnel: w8274 -> [w8297 _]
          tunnel: "Start Saving" -> [_ w8314]
          tunnel: w8269 -> [_ w8313]
          tunnel: [w8296 w8304] -> w8262
          tunnel: w8266 -> [w8296 _]
          tunnel: [w8295 w8303] -> w8263
          tunnel: w8264 -> [w8295 _]
          frame False {
            n1839 = Increment(x=w8302) -> (x+1=w8300:i32)
          }
          frame True {
            w8310 = FALSE ("Start Saving")
            w8315 = 9.0  # File Version
            w8323 = FALSE ("prepend array or string size? (T)")
            w8321 = T31."big-endian, network order" ("byte order (0:big-endian, network order)")
            # "write file headers"
            n1840 = local read "BD 1 Frequency 1 (MHz)"() -> (w8337:dbl)
            n1841 = local read "BD 2 Frequency 1 (MHz)"() -> (w8336:dbl)
            n1842 = local read "BD 1 Frequency 2 (MHz)"() -> (w8335:dbl)
            n1843 = local read "BD 2 Frequency 2 (MHz)"() -> (w8334:dbl)
            n1844 = local read "BD 1 Frequency 3 (MHz)"() -> (w8333:dbl)
            n1845 = local read "BD 2 Frequency 3 (MHz)"() -> (w8332:dbl)
            n1846 = Array Size(array=w8313) -> (size(s)=w8312:i32)
            n1847 = To Double Precision Float(number=w8312) -> (double precision float=w8311:dbl)
            n1848 = local write "Save Calibration"(w8310) -> ()
            n1849 = local write "Start Saving"(w8310) -> ()
            n1850 = Build Array("Save APD Data\nwith Trap Data", "Save Trap Pos. Data") -> (w8307:bool[])
            n1851 = Boolean Array To Number(Boolean array=w8307) -> (number=w8306:u32)
            n1852 = Build Array(w8337, w8336, w8335, w8334, w8333, w8332) -> (w8331:dbl[])
            n1853 = case shown="4" w8341 {
              tunnel: w8340 -> [w8412 w8432 w8448 w8486]
              tunnel: w8311 -> [w8417 w8439 w8468 w8505]
              tunnel: w8338 -> [w8416 w8438 w8467 w8504]
              tunnel: [w8413 w8434 w8459 w8496] -> w8329
              tunnel: [w8404 "Cal sets to save" w8449 w8487] -> w8319
              tunnel: w8331 -> [w8414 w8435 w8461 w8498]
              tunnel: "Save APD Data\nwith Trap Data" -> [w8411 _ w8445 w8484]
              tunnel: [w8411 w8426 w8445 w8484] -> w8316
              tunnel: w8315 -> [w8407 w8427 w8443 w8482]
              tunnel: w8314 -> [w8406 _ _ _]
              tunnel: [w8397 w8426 w8442 w8472] -> w8303
              tunnel: "Save Trap Pos. Data" -> [w8397 _ w8442 w8472]
              tunnel: w8306 -> [w8396 _ w8441 w8471]
              frame 1, Default {
                # "timeseries"
                n1854 = case shown="True" "Profile" {
                  tunnel: [w8420 w8423] -> w8401
                  tunnel: [w8420 w8422] -> w8400
                  tunnel: [w8420 w8421] -> w8399
                  tunnel: [w8420 w8425] -> w8398
                  frame False {
                    w8420 = 0.0 ("f")
                  }
                  frame True {
                    n1855 = local read "Current Position"() -> (w8424:dbl[])
                    n1856 = local read "Y change (mm)"() -> (w8425:dbl)
                    n1857 = call "subVI_explode3array.vi"("Array"=w8424) -> ("x"=w8423:dbl, "y"=w8422:dbl, "z"=w8421:dbl)  [unwired: 12 in]
                  }
                }
                n1858 = local read "Save ave N"() -> (w8419:dbl)
                n1859 = Multiply(x=w8419, y=w8412) -> (x*y=w8418:dbl)
                n1860 = To Double Precision Float(number=w8396) -> (double precision float=w8410:dbl)
                n1861 = Build Array(w8407, w8412, w8418, w8417, w8416, 0.0 ("f")) -> (w8415:dbl[])
                n1862 = Build Array(w8410, w8401, w8400, w8399, w8398) -> (w8408:dbl[])
                n1863 = Select(t=u32 4000000000, s=w8406, f="N sets to save") -> (s? t:f=w8404:u32)
                n1864 = Build Array (concatenate)(w8415, w8414, w8408) -> (w8413:dbl[])
              }
              frame 2 {
                w8429 = 0.0 ("f")
                w8426 = FALSE ("Save APD Data\nwith Trap Data")
                # "calibration"
                n1865 = Boolean To (0,1)(Boolean=w8426) -> (0, 1=w8431:i16)
                n1866 = To Double Precision Float(number=w8431) -> (double precision float=w8430:dbl)
                n1867 = Build Array(w8430, w8429, w8429, w8429, w8429) -> (w8428:dbl[])
                n1868 = Build Array(w8427, w8432, w8432, w8439, w8438, 1.0 ("t")) -> (w8436:dbl[])
                n1869 = Build Array (concatenate)(w8436, w8435, w8428) -> (w8434:dbl[])
                "Calibrating Trap..." <- TRUE ("Calibrating...")
              }
              frame 4 {
                w8446 = 0.0 ("f")
                # "write file header for a trap \nraster scan"
                # "scan dir (x/y = 0/1)"
                # "cycles/step"
                # "n scans (f/b)"
                # "steps"
                # "freq. range"
                # "AOD raster scan"
                n1870 = local read "Number of F/B Scans (AOD)"() -> (w8453:u16)
                n1871 = local read "Cycles/step (AOD)"() -> (w8455:u64)
                n1872 = local read "Scan Range (MHz)"() -> (w8458:dbl)
                n1873 = local read "Scan steps (AOD)"() -> (w8457:u64)
                n1874 = local read "Scan BD"() -> (w8465:bool)
                n1875 = local read "Save ave N"() -> (w8470:dbl)
                n1876 = Boolean To (0,1)(Boolean=w8465) -> (0, 1=w8464:i16)
                n1877 = To Double Precision Float(number=w8453) -> (double precision float=w8452:dbl)
                n1878 = To Double Precision Float(number=w8457) -> (double precision float=w8456:dbl)
                n1879 = To Double Precision Float(number=w8455) -> (double precision float=w8454:dbl)
                n1880 = To Double Precision Float(number=w8464) -> (double precision float=w8463:dbl)
                n1881 = Multiply(x=w8470, y=w8448) -> (x*y=w8469:dbl)
                n1882 = To Double Precision Float(number=w8441) -> (double precision float=w8447:dbl)
                n1883 = Build Array(w8447, w8446, w8446, w8446, w8446) -> (w8444:dbl[])
                n1884 = local read "N sets should be saved"() -> (w8450:dbl)
                n1885 = Build Array(w8463, w8458, w8456, w8454, w8452) -> (w8460:dbl[])
                n1886 = Build Array(w8443, w8448, w8469, w8468, w8467, 2.0 ("t")) -> (w8462:dbl[])
                n1887 = Round Toward +Infinity(x=w8450) -> (ceil(x): smallest int >= x=w8451:dbl)
                n1888 = Build Array (concatenate)(w8462, w8461, w8444, w8460) -> (w8459:dbl[])
                n1889 = To Unsigned Long Integer(number=w8451) -> (unsigned 32bit integer=w8449:u32)
              }
              frame 8 {
                w8479 = 0.0 ("f")
                # "MCL raster scan"
                n1890 = local read "Number of scans (MCL)"() -> (w8474:u64)
                n1891 = local read "Scan lines (y)"() -> (w8473:u64)
                n1892 = local read "2D or 1D Scan"() -> (w8476:bool)
                n1893 = local read "Scan Range (V)\n(of steps)"() -> (w8495:dbl)
                n1894 = local read "Fast Scan Dir"() -> (w8502:bool)
                n1895 = local read "Cycles/step (MCL)"() -> (w8492:u64)
                n1896 = local read "Scan steps (MCL)"() -> (w8494:u64)
                n1897 = Select(t=w8473, s=w8476, f=w8474) -> (s? t:f=w8475:u64)
                n1898 = Boolean To (0,1)(Boolean=w8476) -> (0, 1=w8478:i16)
                n1899 = local read "Save ave N"() -> (w8507:dbl)
                n1900 = local read "Initial X"() -> (w8481:dbl)
                n1901 = local read "Initial Y"() -> (w8480:dbl)
                n1902 = To Double Precision Float(number=w8478) -> (double precision float=w8477:dbl)
                n1903 = Boolean To (0,1)(Boolean=w8502) -> (0, 1=w8501:i16)
                n1904 = To Double Precision Float(number=w8475) -> (double precision float=w8490:dbl)
                n1905 = To Double Precision Float(number=w8494) -> (double precision float=w8493:dbl)
                n1906 = To Double Precision Float(number=w8492) -> (double precision float=w8491:dbl)
                n1907 = To Double Precision Float(number=w8501) -> (double precision float=w8500:dbl)
                n1908 = Multiply(x=w8507, y=w8486) -> (x*y=w8506:dbl)
                n1909 = To Double Precision Float(number=w8471) -> (double precision float=w8485:dbl)
                n1910 = local read "N sets should be saved (MCL)"() -> (w8488:dbl)
                n1911 = Build Array(w8485, w8477, w8479, w8479, w8479) -> (w8483:dbl[])
                n1912 = Build Array(w8500, w8495, w8493, w8491, w8490, w8481, w8480) -> (w8497:dbl[])
                n1913 = Build Array(w8482, w8486, w8506, w8505, w8504, 3.0 ("t")) -> (w8499:dbl[])
                n1914 = Round Toward +Infinity(x=w8488) -> (ceil(x): smallest int >= x=w8489:dbl)
                n1915 = Build Array (concatenate)(w8499, w8498, w8483, w8497) -> (w8496:dbl[])
                n1916 = To Unsigned Long Integer(number=w8489) -> (unsigned 32bit integer=w8487:u32)
              }
            }
            n1917 = local read "Index"() -> (w8346:dbl)
            n1918 = call "Create new save file.vi"("Insert"="", "Ext"=".dat", "Index In"=w8346) -> ("Path Out"=w8305:path, "Index Out"=w8318:dbl)
            n1919 = local write "Save file name"(w8305) -> ()
            n1920 = local write "Index"(w8318) -> ()
            n1921 = local write "Save index"(w8318) -> ()
            n1922 = Array Size(array=w8329) -> (size(s)=w8330:i32)
            n1923 = Open/Create/Replace File(file path (use dialog)=w8305, operation (0:open)=T25."create", access (0:read/write)=enum16{"read/write", "read-only", "write-only"}."write-only") -> (refnum out=w8343:refnum<file>)  [unwired: 1 in, 4 out]
            n1924 = local write "Saving..."(TRUE ("Saving...")) -> ()
            n1925 = To Double Precision Float(number=w8330) -> (double precision float=w8328:dbl)
            n1926 = String Length(string="Comment (data description)") -> (length=w8326:i32)
            n1927 = To Double Precision Float(number=w8326) -> (double precision float=w8325:dbl)
            n1928 = Deny Access(7:w8343) -> (3:w8342:refnum<file>)  [unwired: 1 in, 2 out]
            n1929 = Build Array (concatenate)(w8328, w8329, w8325) -> (w8327:dbl[])
            n1930 = case "If fluorescence data to be saved" shown="True" w8316 {
              tunnel: w8305 -> [_ w8395]
              tunnel: [refnum<k0> refnum w8375] -> w8317
              frame False {
              }
              frame True {
                w8374 = 0.0
                n1931 = local read "APD Integration Time (s)"() -> (w8380:dbl)
                n1932 = local read "N APD Samp/step"() -> (w8373:dbl)
                n1933 = Path To String(path=w8395) -> (string=w8394:string)
                n1934 = String Length(string=w8394) -> (length=w8393:i32)
                n1935 = Subtract(x=w8393, y=4) -> (x-y=w8391:i32)
                n1936 = String Subset(string=w8394, length (rest)=w8391) -> (substring=w8390:string)  [unwired: 1 out]
                n1937 = Build Array(w8380, w8373, w8374, w8374, w8374, w8374, w8374, w8374) -> (w8377:dbl[])
                n1938 = Concatenate Strings(w8390, "_fl.dat" ("string")) -> (w8388:string)
                n1939 = Array Size(array=w8377) -> (size(s)=w8379:i32)
                n1940 = String To Path(string=w8388) -> (path=w8384:path)
                n1941 = Open/Create/Replace File(file path (use dialog)=w8384, operation (0:open)=T25."create", access (0:read/write)=enum16{"read/write", "read-only", "write-only"}."write-only") -> (refnum out=w8385:refnum<file>)  [unwired: 1 in, 4 out]
                n1942 = Deny Access(7:w8385) -> (3:w8381:refnum<file>)  [unwired: 1 in, 2 out]
                n1943 = To Double Precision Float(number=w8379) -> (double precision float=w8378:dbl)
                n1944 = Build Array (concatenate)(w8378, w8377) -> (w8376:dbl[])
                n1945 = Write to Binary File(file (use dialog)=w8381, data=w8376, 5:FALSE ("prepend array or string size? (T)"), 9:T31."big-endian, network order" ("byte order (0:big-endian, network order)")) -> (refnum out=w8375:refnum<file>)  [unwired: 1 in, 3 out]
              }
            }
            n1946 = case shown="True" w8303 {
              tunnel: w8305 -> [_ w8357]
              tunnel: [refnum<k0> refnum w8356] -> w8304
              frame False {
              }
              frame True {
                w8352 = 0.0 ("element")
                n1947 = Path To String(path=w8357) -> (string=w8371:string)
                n1948 = Build Array(w8352, w8352, w8352, w8352, w8352, w8352, w8352, w8352) -> (w8353:dbl[])
                n1949 = String Length(string=w8371) -> (length=w8370:i32)
                n1950 = Subtract(x=w8370, y=4) -> (x-y=w8368:i32)
                n1951 = Array Size(array=w8353) -> (size(s)=w8355:i32)
                n1952 = String Subset(string=w8371, length (rest)=w8368) -> (substring=w8367:string)  [unwired: 1 out]
                n1953 = To Double Precision Float(number=w8355) -> (double precision float=w8354:dbl)
                n1954 = Concatenate Strings(w8367, "_pos.dat" ("string")) -> (w8365:string)
                n1955 = Build Array (concatenate)(w8354, w8353) -> (w8351:dbl[])
                n1956 = String To Path(string=w8365) -> (path=w8361:path)
                n1957 = Open/Create/Replace File(file path (use dialog)=w8361, operation (0:open)=T25."create", access (0:read/write)=enum16{"read/write", "read-only", "write-only"}."write-only") -> (refnum out=w8362:refnum<file>)  [unwired: 1 in, 4 out]
                n1958 = Deny Access(7:w8362) -> (3:w8358:refnum<file>)  [unwired: 1 in, 2 out]
                n1959 = Write to Binary File(file (use dialog)=w8358, data=w8351, 5:FALSE ("prepend array or string size? (T)"), 9:T31."big-endian, network order" ("byte order (0:big-endian, network order)")) -> (refnum out=w8356:refnum<file>)  [unwired: 1 in, 3 out]
              }
            }
            n1960 = Write to Binary File(file (use dialog)=w8342, data=w8327, 5:w8323, 9:w8321) -> (refnum out=w8324:refnum<file>)  [unwired: 1 in, 3 out]
            n1961 = Write to Binary File(file (use dialog)=w8324, data="Comment (data description)", 5:w8323, 9:w8321) -> (refnum out=w8320:refnum<file>)  [unwired: 1 in, 3 out]
          }
        }
        n1962 = feedback-in #19(w8263) -> ()
        n1963 = feedback-in #20(w8290) -> ()
        n1964 = feedback-in #21(w8262) -> ()
        n1965 = feedback-in #22(w8273) -> ()
        n1966 = feedback-in #23(w8276) -> ()
        n1967 = feedback-in #24(w8289) -> ()
        n1968 = feedback-in #25(w8279) -> ()
      }
      frame #1 {
        n1969 = local read "Saving..."() -> (w8520:bool)
        n1970 = case shown="True" w8520 {
          tunnel: w8524 -> [_ w8534]
          tunnel: w8523 -> [_ w8548]
          tunnel: w8522 -> [_ w8544]
          tunnel: w8521 -> [_ w8543]
          tunnel: w8519 -> [_ w8542]
          tunnel: w8518 -> [_ w8537]
          tunnel: w8517 -> [_ w8536]
          tunnel: w8516 -> [_ w8535]
          tunnel: w8515 -> [_ w8533]
          tunnel: w8514 -> [_ w8531]
          tunnel: w8513 -> [_ w8530]
          tunnel: w8512 -> [_ w8529]
          tunnel: w8511 -> [_ w8528]
          tunnel: w8510 -> [_ w8527]
          tunnel: w8509 -> [_ w8526]
          tunnel: w8508 -> [_ w8525]
          frame False {
          }
          frame True {
            n1971 = Multiply(x=w8534, y=w8533) -> (x*y=→"Time (s)":dbl)
            n1972 = Less Or Equal?(x=w8534, y=w8542) -> (x <= y?=w8546:bool)
            n1973 = Or(x="Stop Saving", y="Abort save 2") -> (x .or. y?=w8538:bool)
            n1974 = Not(x=w8538) -> (.not. x?=w8547:bool)
            n1975 = And(x=w8546, y=w8547) -> (x .and. y?=w8545:bool)
            n1976 = case shown="False" w8545 {
              tunnel: w8548 -> [w8555 w8623]
              tunnel: [0.0 w8626] -> w8541
              tunnel: w8534 -> [_ w8624]
              tunnel: w8542 -> [_ w8625]
              tunnel: w8544 -> [_ w8620]
              tunnel: w8543 -> [_ _]
              tunnel: w8537 -> [w8553 w8613]
              tunnel: w8536 -> [w8552 w8614]
              tunnel: w8535 -> [_ w8612]
              tunnel: w8531 -> [_ w8611]
              tunnel: w8530 -> [_ w8565]
              tunnel: w8529 -> [_ w8604]
              tunnel: w8528 -> [_ w8582]
              tunnel: w8527 -> [w8550 w8563]
              tunnel: w8526 -> [w8551 w8562]
              tunnel: w8525 -> [_ w8559]
              frame False {
                w8549 = FALSE
                n1977 = Close File(refnum=w8555) -> ()  [unwired: 1 in, 2 out]